vi "Main1.vi"() -> ()   [LabVIEW 2020]
uses:
  System.Windows.Forms
  Global_Variable/Global.vi
  Database/Global1.vi
  <userlib>/_MGI/Menu Building/MenuTypes/MenuStrip/MGI_MenuStrip.lvclass
  <userlib>/_MGI/Menu Building/MenuItemStatusChange/MGI_MenuItemStatusChange.lvclass
  Libraries/S7/S7.lvlib
panel:
  in  "Andon":enum32{"未选择", "缺料报警", "质量报警", "故障报警"}(radio)
  out "自动":bool
  out "结果显示":string
  in  "打印条码":bool caption="布尔"
  out "传感器值":dbl format="%#_4gN"
  out "上学状态":string="123"
  out "PLC":bool
  in  "菜单":refnum<k24>(container)
  out "试验计时":u16
  out "产品编号":string
  out "生产数量":i32
  out "合格数量":i32
  out "userStatus":string caption="用户状态"
  out "userName":string caption="用户名"
  out "connectionMode":string caption="联机类型"
  out "产品型号":string
  out "锁紧/开启":bool
  in  "更换产品":refnum<vi>
  out "提示信息":string
  out "错误":bool
  out "时间字符串":string
  out "日期字符串":string
  # "中间轴装配"
  # "装配工艺"
  # "上序状态"
  # "检测结果："
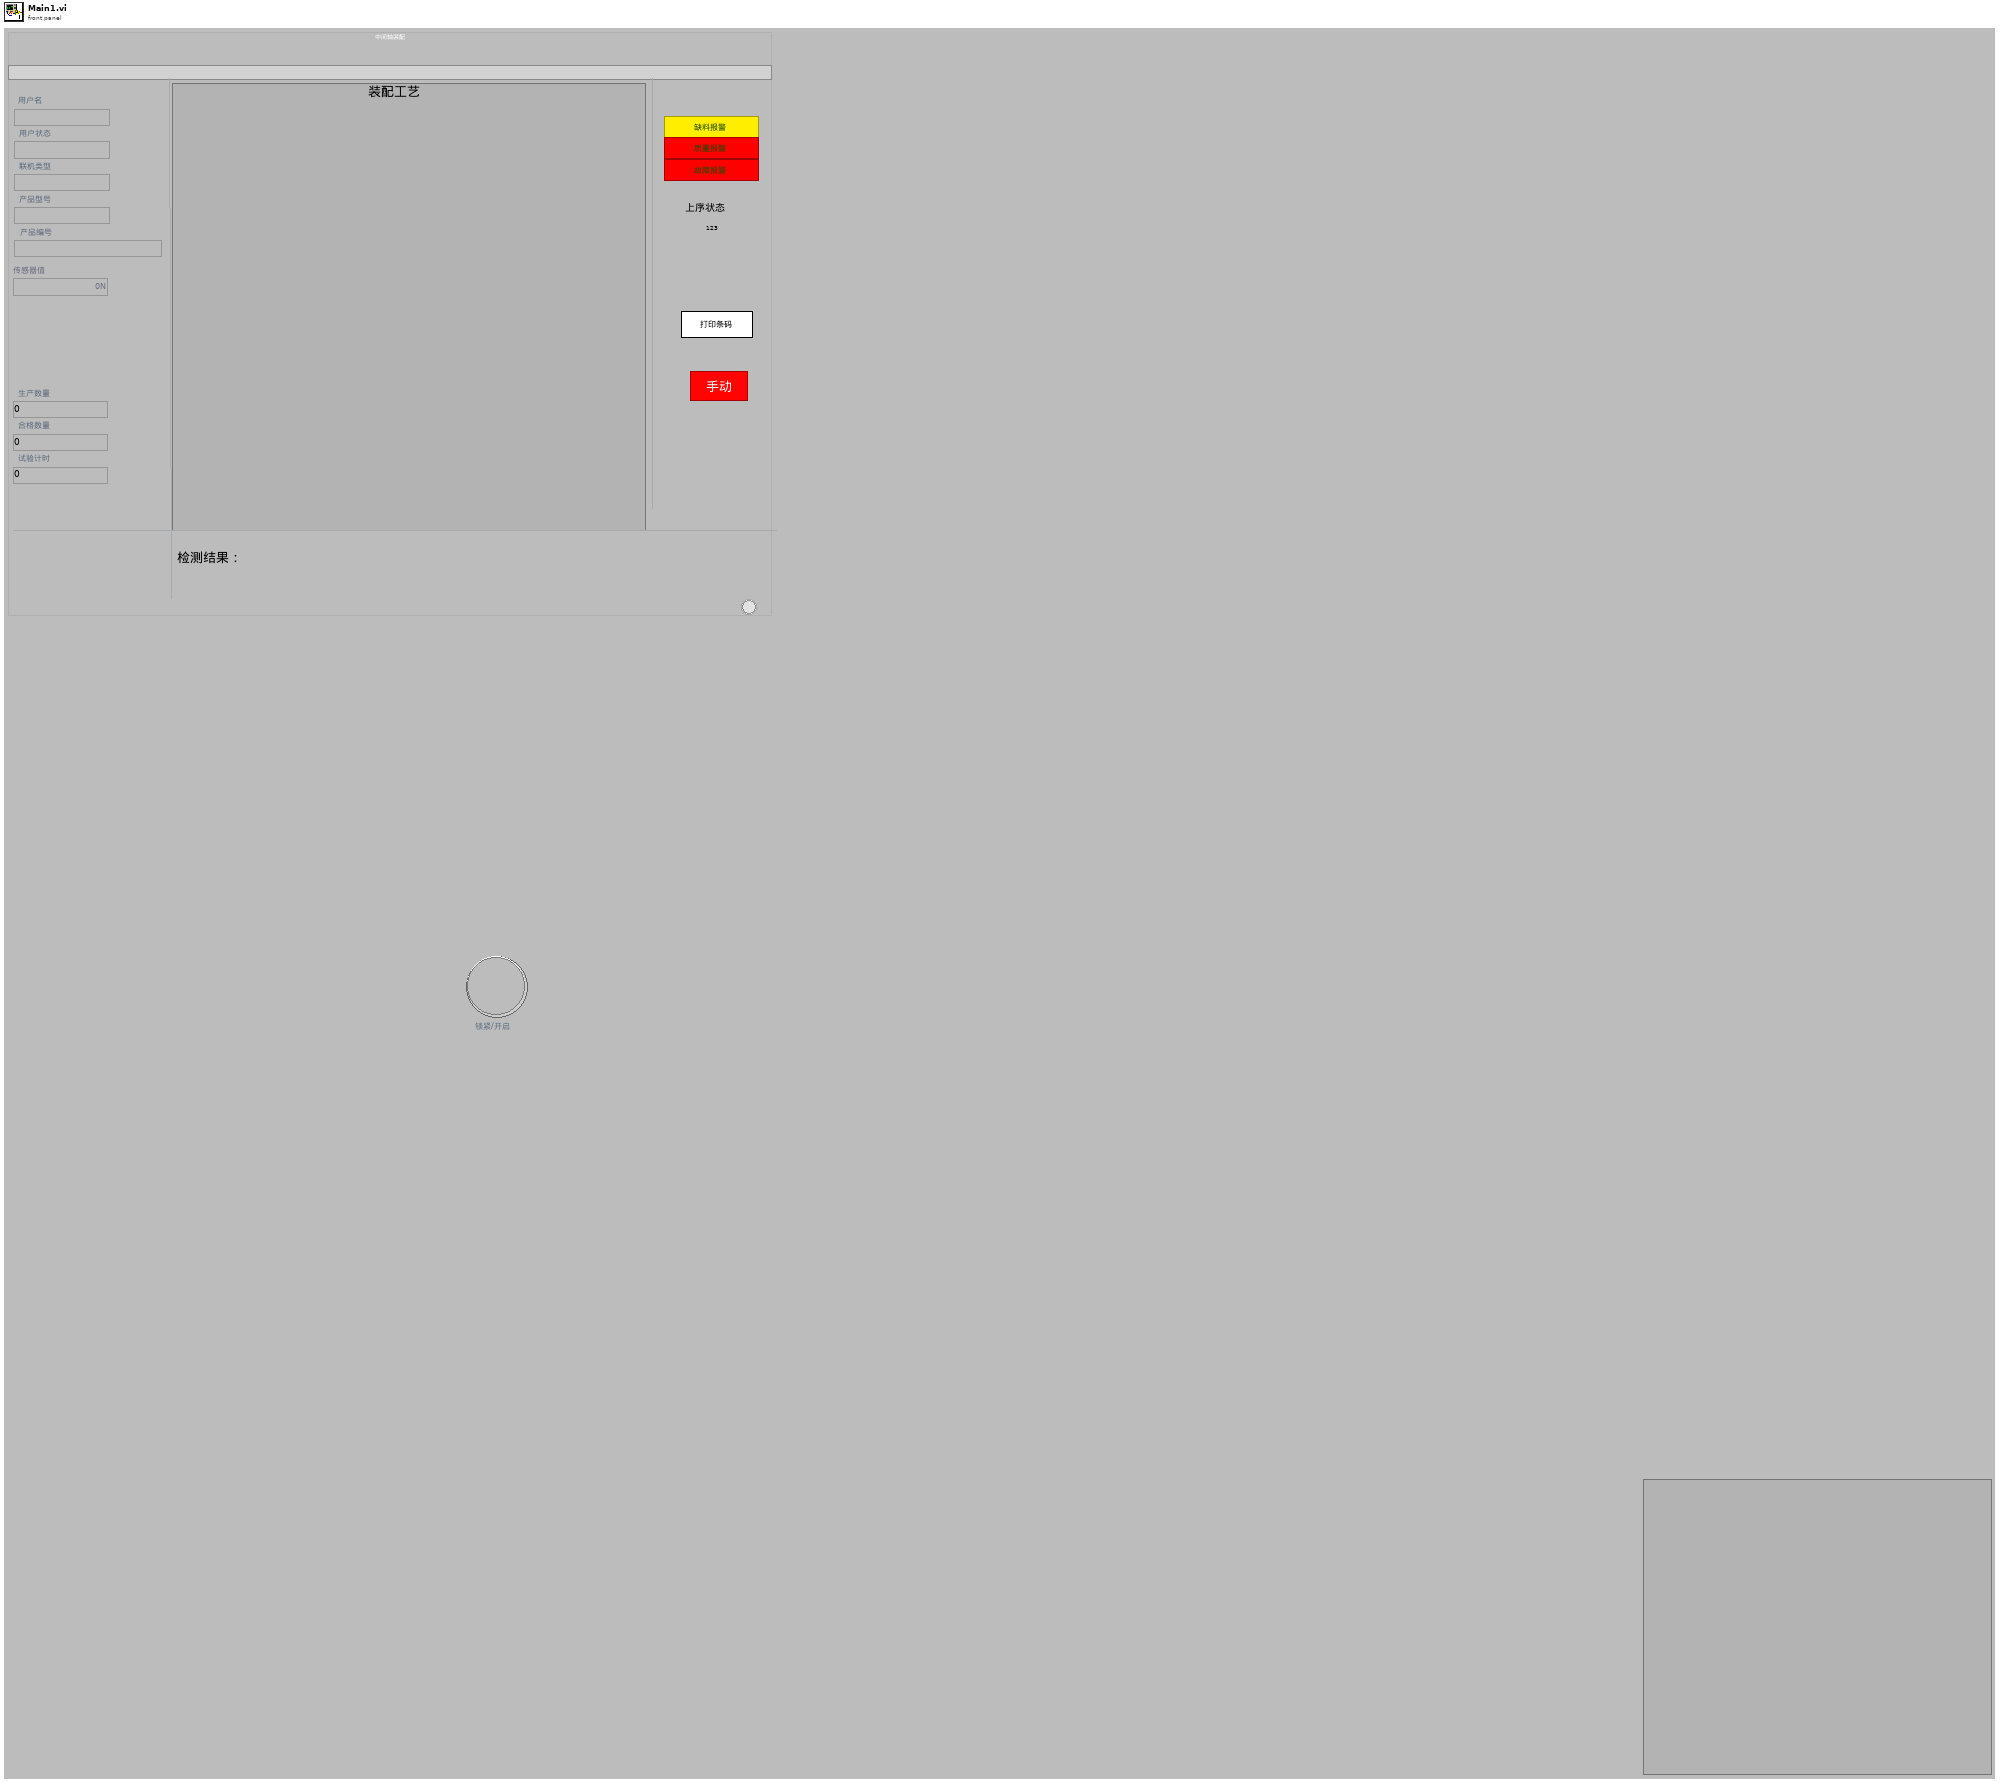
[diagram p1: front panel]
types:
  T1 = typedef "S7.lvlib/Broadcast Events--cluster.ctl" = cluster{"Module Did Init":refnum<user-event>, "Status Updated":refnum<user-event>, "Error Reported":refnum<user-event>, "Module Did Stop":refnum<user-event>, "Update Module Execution Status":refnum<user-event>}
  T2 = enum32{"Invalid", "Standard", "Closed", "Hidden", "Minimized", "Maximized"}
  T3 = cluster{"设备名称":string, "操作人员":string, "设备状态":enum16{"设备离线", "设备正常", "设备缺料", "设备故障", "质量报警"}, "附加信息":string}
  T4 = enum32{"invalid app kind", "Development System", "Run Time System", "Student Edition", "Embedded LabVIEW", "Evaluation", "Custom"}
  T5 = cluster{"扭矩":sgl, "输入移载位移":sgl, "工装移载位移":sgl, "输入编码位移":sgl, "输入扭矩":sgl, "输出扭矩(小)":sgl, "输出扭矩(大)":sgl, "吸收电流":sgl}
  T6 = cluster{"用户编号":string, "用户名":string, "用户密码(密文)":string, "用户权限":string}
  T7 = cluster{"Core":cluster{"Current VI Reference":refnum<vi>, "Close Panel on Exit?":bool}, "Your Boolean data":bool, "Your string data":string}
  T8 = enum32{"Bad", "Idle", "Run top level", "Running"}
  T9 = cluster{"Current VI Reference":refnum<vi>, "Close Panel on Exit?":bool}
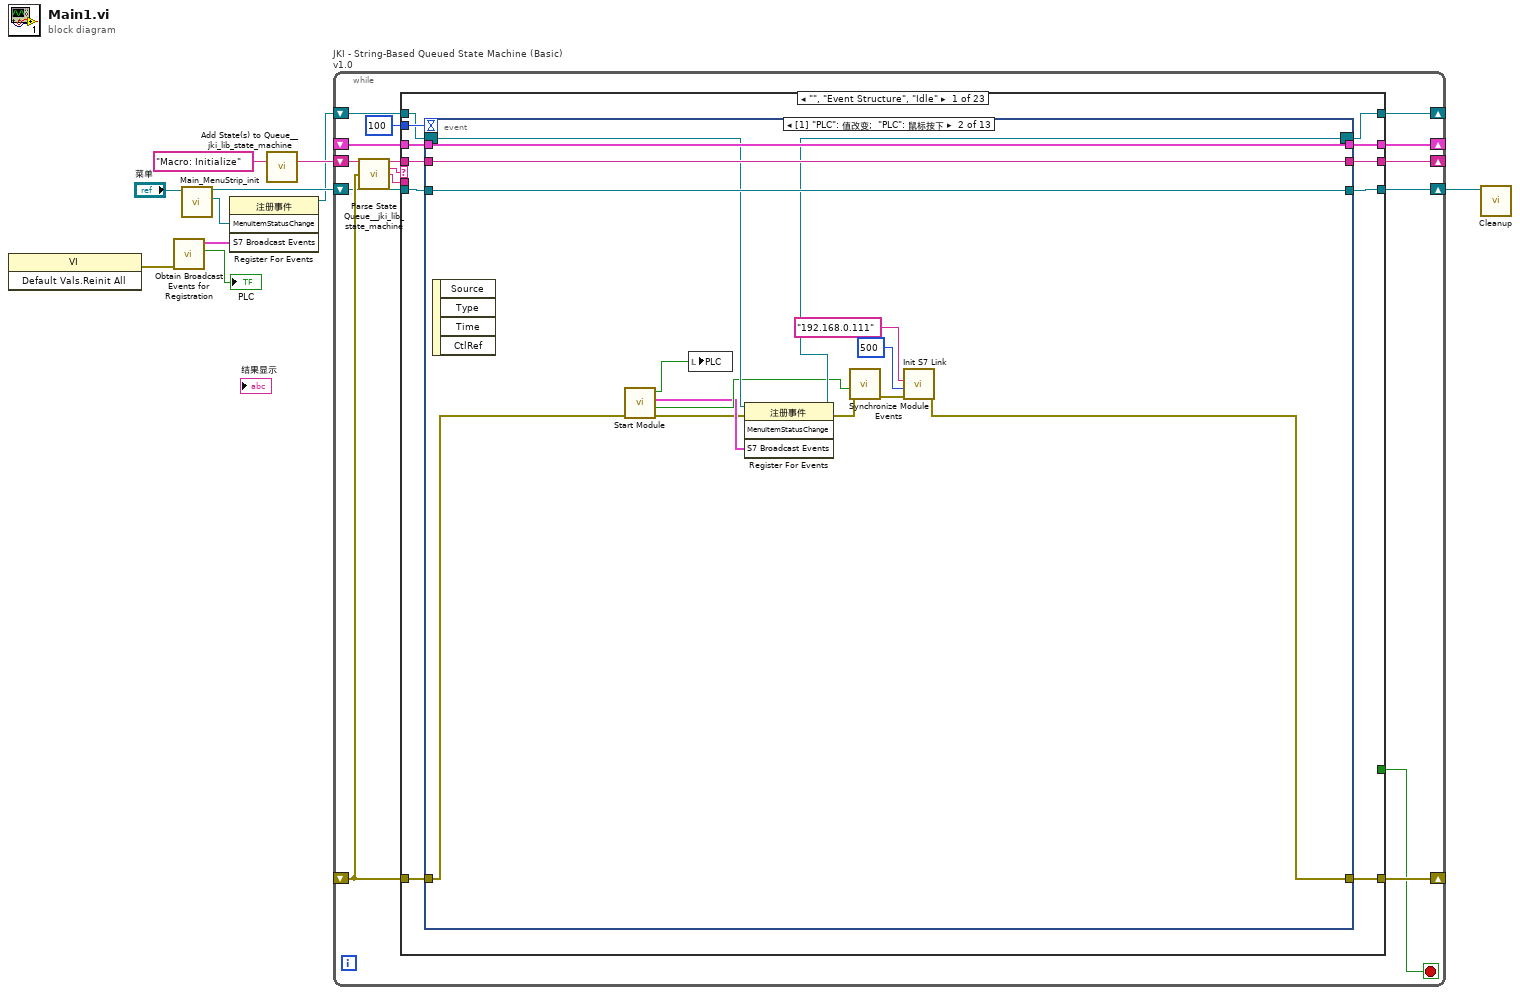
[diagram p0: block diagram]
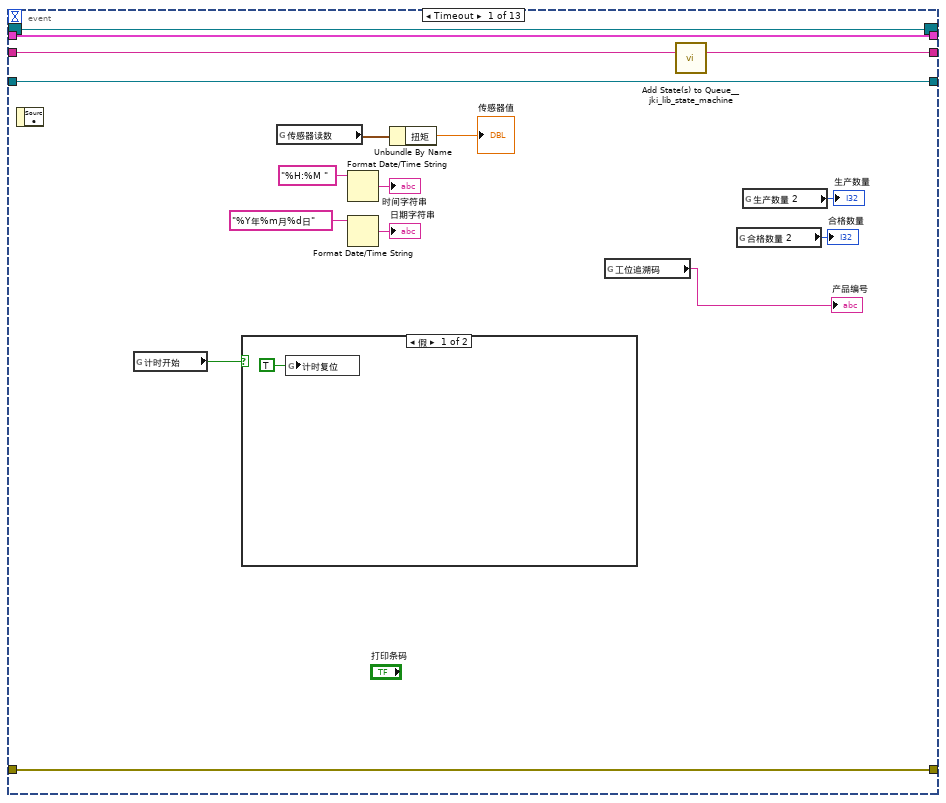
[diagram p2: hidden frame]
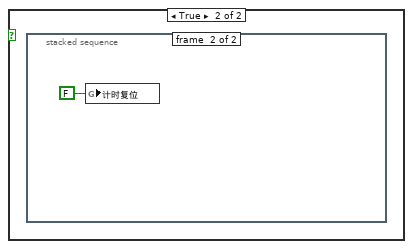
[diagram p3: hidden frame]
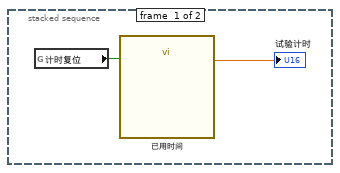
[diagram p4: hidden frame]
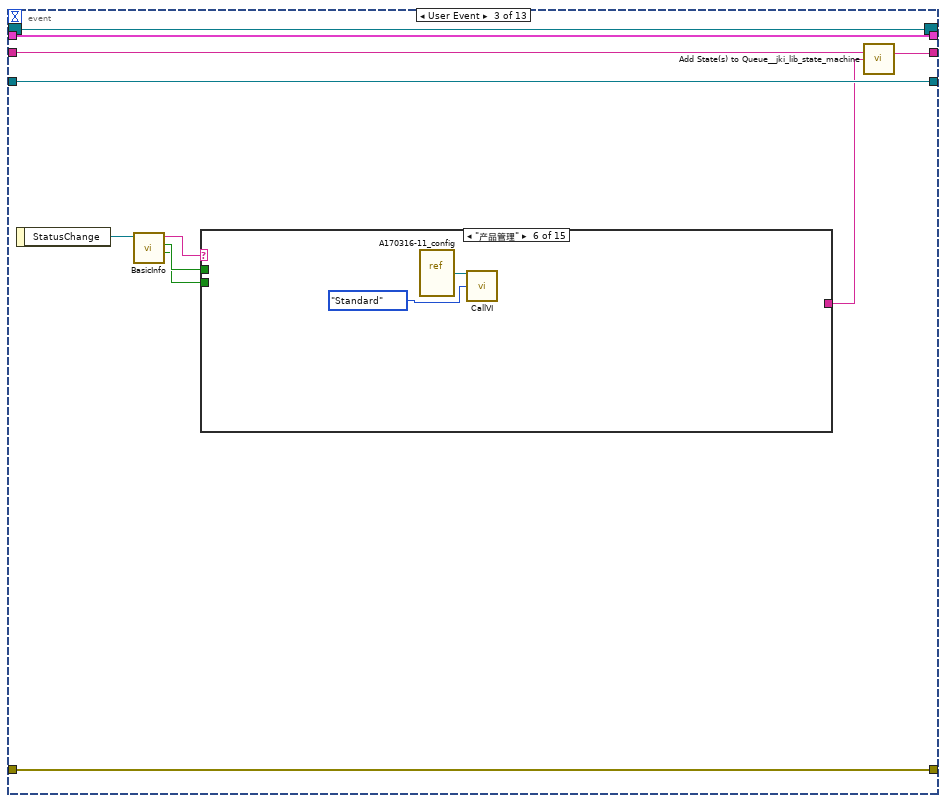
[diagram p5: hidden frame]
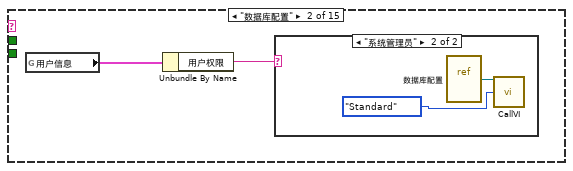
[diagram p7: hidden frame]
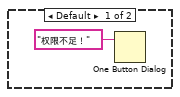
[diagram p8: hidden frame]
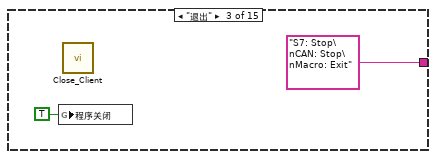
[diagram p9: hidden frame]
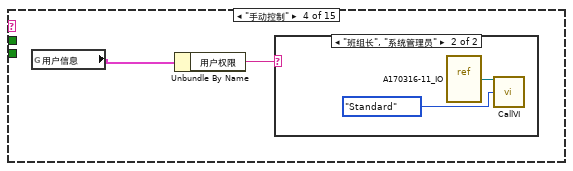
[diagram p10: hidden frame]
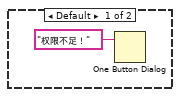
[diagram p11: hidden frame]
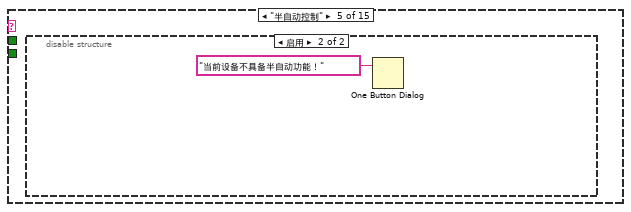
[diagram p12: hidden frame]
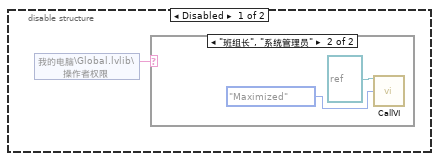
[diagram p13: hidden frame]
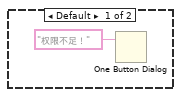
[diagram p14: hidden frame]
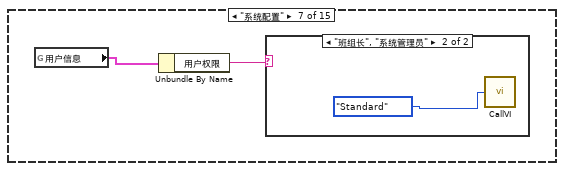
[diagram p15: hidden frame]
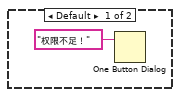
[diagram p16: hidden frame]
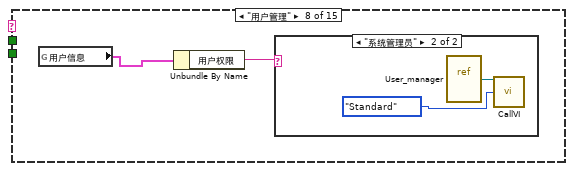
[diagram p17: hidden frame]
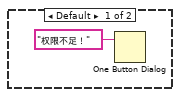
[diagram p18: hidden frame]
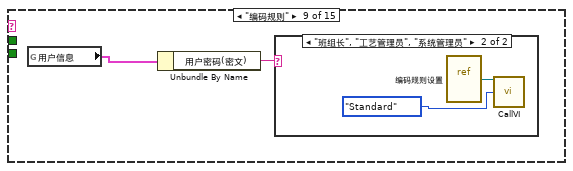
[diagram p19: hidden frame]
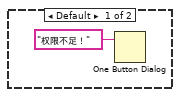
[diagram p20: hidden frame]
diagram:
  n1 = invoke class="VI" method="Default Vals.Reinit All"() -> (error out=w3:errorcluster)  [unwired: 3 in, 2 out]
  n2 = call "Obtain Broadcast Events for Registration.vi"("error in (no error)"=w3) -> ("Already running?"=→"PLC":bool, "S7 Broadcast Events"=w5:T1)  [unwired: 8 in, 1 out]
  n3 = call "Main_MenuStrip_init.vi"("MenuStrip"="菜单") -> ("MenuItemStatusChange"=w2:refnum<user-event>, "Menu out"=w7:refnum<class "MGI_MenuStrip.lvclass">)  [unwired: 9 in]
  n4 = register-events(w2, w5) -> (reference out=w1:refnum<event-registration>)  [unwired: 2 in, 1 out]
  n5 = call <vilib>:"Add State(s) to Queue__jki_lib_state_machine.vi"("State(s) in (\"\")"="Macro: Initialize") -> ("States Out"=w10:string)  [unwired: 14 in]
  n6 = while "JKI - String-Based Queued State Machine (Basic) v1.0" {
    shift-right: [w19] -> _
    shift-left: _ -> [w18]
    shift-right: [w21] -> _
    shift-left: _ -> [w16]
    shift-right: [w20] -> _
    shift-left: w10 -> [w22]
    shift-right: [w14] -> w6
    shift-left: w7 -> [w15]
    shift-right: [w12] -> _
    shift-left: w1 -> [w11]
    stop <- w13 stop-if-true
    n7 = call <vilib>:"Parse State Queue__jki_lib_state_machine.vi"("State Queue"=w22, "Error In (no error)"=w16) -> ("Remaining States"=w24:string, "Current State"=w25:string, "Arguments"=w23:string)  [unwired: 11 in]
    n8 = case shown="\"\", \"Event Structure\", \"Idle\"" w25 {
      selector: w25 -> [_ _ w242 _ _ _ _ _ _ _ _ _ _ _ _ _ _ _ _ _ _ _ _]
      tunnel: w24 -> [w36 w239 w246 w266 w274 w281 w287 w291 w297 w303 w324 w333 w344 w352 w358 w365 w392 w422 w430 w443 w471 w478 w490]
      tunnel: w23 -> [_ _ _ _ _ _ _ _ _ _ _ _ _ _ _ _ _ _ w425 w437 _ _ _]
      tunnel: w18 -> [w34 w236 w244 w257 w271 w279 w284 w292 w300 w306 w327 w330 _ w347 w355 w363 w390 w419 w428 w439 w468 w475 w487]
      tunnel: [w33 w237 w248 w263 errorcluster {"status"=FALSE, "code"=0, "source"=""} ("error out") w278 w285 w289 w295 w302 w323 w331 w341 w348 w356 w362 w388 w420 w426 w440 w469 w476 w488] -> w21
      tunnel: w16 -> [w32 w237 w247 w263 w270 w278 w285 w289 w296 w302 w323 w331 w341 w349 w356 w359 w388 w420 w427 w441 w469 w476 w488]
      tunnel: [w35 w238 w245 w265 w273 w280 w286 w291 w298 w304 w325 w332 w343 w351 w357 w364 w391 w421 w429 w442 w470 w477 w489] -> w20
      tunnel: [w31 w236 w244 w264 w271 w279 w284 w292 w300 w306 w327 w330 w342 w347 w355 w363 w390 w419 w428 w439 w468 w475 w487] -> w19
      tunnel: 100 ("Timeout") -> [w30 _ _ _ _ _ _ _ _ _ _ _ _ _ _ _ _ _ _ _ _ _ _]
      tunnel: w15 -> [w29 w235 w241 w254 w268 w277 w283 w290 w299 w305 w326 w329 w335 w346 w354 w361 w389 w418 w424 w436 w467 w473 w480]
      tunnel: [w28 w235 w241 w254 w268 w277 w283 w290 w299 w305 w326 w329 w335 w346 w354 w361 w389 w418 w424 w436 w467 w473 w480] -> w14
      tunnel: [_ _ _ _ _ TRUE _ _ _ _ _ _ _ _ _ _ _ _ _ _ _ _ _] -> w13
      tunnel: [w26 w234 w240 w253 w267 w275 w282 w293 w294 w301 w322 w328 w336 w345 w353 w360 w387 w415 w423 w435 w466 w472 w479] -> w12
      tunnel: w11 -> [w27 w234 w240 w253 w267 w275 w282 w293 w294 w301 w322 w328 w336 w345 w353 w360 w387 w415 w423 w435 w466 w472 w479]
      frame "", "Event Structure", "Idle" {
        n9 = event shown="[1] \"PLC\": 值改变;  \"PLC\": 鼠标按下" {
          selector: w27 -> [w41 w66 w72 w137 w144 w151 w158 w173 w188 w190 w197 w206 _]
          dyn-events: [w41 w65 w72 w137 w144 w151 w158 w173 w188 w190 w197 w206 _] -> w26
          timeout: w30 -> [_ _ _ _ _ _ _ _ _ _ _ _ _]
          tunnel: w36 -> [w52 w70 w81 w138 w145 w154 w161 w170 w186 w194 w204 w208 w228]
          tunnel: [w51 w70 w79 w139 w146 w155 w162 w171 w186 w195 w203 w209 w228] -> w35
          tunnel: w34 -> [w50 w71 w80 w141 w149 w156 w163 w172 w187 w196 w201 w211 w229]
          tunnel: [w42 w67 w82 w142 w147 w152 w164 w168 w184 w193 w202 w210 w226] -> w33
          tunnel: w32 -> [w42 w68 w82 w142 w147 w152 w165 w168 w184 w193 w202 w210 w226]
          tunnel: [w50 w71 w80 w141 w149 w156 w163 w172 w187 w196 w201 w211 w229] -> w31
          tunnel: w29 -> [w40 w69 w75 w140 w148 w153 w160 w169 w185 _ _ _ w227]
          tunnel: [w40 w69 w75 w140 w148 w153 w160 w169 w185 _ _ _ w227] -> w28
          event Timeout {
            n10 = event-data() -> ()  [unwired: 1 in, 1 out]
            n11 = global read "Global.vi" "计时开始"() -> (w43:bool)
            n12 = case shown="假" w43 {
              frame False {
                n13 = global write "Global.vi" "计时复位"(TRUE ("计时复位")) -> ()
              }
              frame True {
                n14 = stacked-sequence {
                  frame #0 {
                    n15 = global read "Global.vi" "计时复位"() -> (w54:bool)
                    n16 = call "已用时间"("Reset"=w54) -> ("Elapsed Time (s)"=→"试验计时":dbl)  [unwired: 11 in, 7 out]
                  }
                  frame #1 {
                    n17 = global write "Global.vi" "计时复位"(FALSE ("计时复位")) -> ()
                  }
                }
              }
            }
            n18 = global read "Global.vi" "传感器读数"() -> (w38:T5)
            n19 = Format Date/Time String(time format string (%c)="%H:%M ") -> (date/time string=→"时间字符串":string)  [unwired: 2 in]
            n20 = Format Date/Time String(time format string (%c)="%Y年%m月%d日") -> (date/time string=→"日期字符串":string)  [unwired: 2 in]
            n21 = Unbundle By Name(w38) -> ("扭矩"=→"传感器值":sgl)
            n22 = global read "Global1.vi" "工位追溯码"() -> (→"产品编号":string)
            n23 = call <vilib>:"Add State(s) to Queue__jki_lib_state_machine.vi"("State(s) in (\"\")"=w52) -> ("States Out"=w51:string)  [unwired: 14 in]
            n24 = global read "Global.vi" "合格数量 2"() -> (→"合格数量":i32)
            n25 = global read "Global.vi" "生产数量 2"() -> (→"生产数量":i32)
          }
          event "PLC": Value Change; "PLC": Mouse Down {
            n26 = event-data() -> ()  [unwired: 1 in, 4 out]
            n27 = call "Start Module.vi"("error in (no error)"=w68) -> ("error out"=w61:errorcluster, "Wait for Event Sync?"=w64:bool, "S7 Broadcast Events"=w63:T1, "Module Was Already Running?"=w62:bool)  [unwired: 7 in]
            n28 = local write "PLC"(w62) -> ()
            n29 = register-events(reference=w66, error in=w61, w63) -> (reference out=w65:refnum<event-registration>, error out=w60:errorcluster)  [unwired: 1 in]
            n30 = call "Synchronize Module Events.vi"("error in (no error)"=w60, "Wait for Event Sync?"=w64) -> ("error out"=w57:errorcluster)  [unwired: 9 in]
            n31 = call "Init S7 Link.vi"("error in (no error)"=w57, "超时"=500, "IP"="192.168.0.111") -> ("error out"=w67:errorcluster)  [unwired: 8 in]
          }
          event User Event {
            n32 = event-data() -> ("StatusChange"=w73:refnum<class "MGI_MenuItemStatusChange.lvclass">)  [unwired: 1 in]
            n33 = call <userlib>:"BasicInfo.vi"("MGI_MenuItemStatusChange in"=w73) -> ("Enabled?"=w76:bool, "Checked?"=w77:bool, "Tag"=w78:string)  [unwired: 7 in, 1 out]
            n34 = case shown="\"产品管理\"" w78 {
              tunnel: w77 -> [_ _ _ _ _ _ _ _ _ _ _ _ _ _ _]
              tunnel: w76 -> [_ _ _ _ _ _ _ _ _ _ _ _ _ _ _]
              tunnel: [_ _ "S7: Stop\nCAN: Stop\nMacro: Exit" _ _ _ _ _ _ _ _ _ _ _ _] -> w74
              frame "假", Default {
              }
              frame "数据库配置" {
                n35 = global read "Global1.vi" "用户信息"() -> (w83:T6)
                n36 = Unbundle By Name(w83) -> ("用户权限"=w84:string)
                n37 = case shown="\"系统管理员\"" w84 {
                  frame Default {
                    n38 = One Button Dialog(message="权限不足！" ("消息")) -> ()  [unwired: 1 in, 1 out]
                  }
                  frame "系统管理员" {
                    n39 = vi-ref "数据库配置.vi"() -> (w87:refnum<vi>)
                    n40 = call "CallVI.vi"("VI引用"=w87, "状态"=T2."Standard") -> ()  [unwired: 11 in, 3 out]
                  }
                }
              }
              frame "退出" {
                n41 = global write "Global.vi" "程序关闭"(TRUE ("程序关闭")) -> ()
                n42 = call "Close_Client.vi"() -> ()  [unwired: 12 in]
              }
              frame "手动控制" {
                n43 = global read "Global1.vi" "用户信息"() -> (w90:T6)
                n44 = Unbundle By Name(w90) -> ("用户权限"=w91:string)
                n45 = case shown="\"班组长\", \"系统管理员\"" w91 {
                  frame Default {
                    n46 = One Button Dialog(message="权限不足！" ("消息")) -> ()  [unwired: 1 in, 1 out]
                  }
                  frame "班组长", "系统管理员" {
                    n47 = vi-ref "A170316-11_IO.vi"() -> (w94:refnum<vi>)
                    n48 = call "CallVI.vi"("VI引用"=w94, "状态"=T2."Standard") -> ()  [unwired: 11 in, 3 out]
                  }
                }
              }
              frame "半自动控制" {
                n49 = disable-structure shown="启用" {
                  frame Disabled {
                    n50 = shared-variable "我的电脑\\Global.lvlib\\操作者权限"() -> (w95:string)  [unwired: 1 in, 1 out]
                    n51 = case shown="\"班组长\", \"系统管理员\"" w95 {
                      frame Default {
                        n52 = One Button Dialog(message="权限不足！" ("消息")) -> ()  [unwired: 1 in, 1 out]
                      }
                      frame "班组长", "系统管理员" {
                        n53 = call "CallVI.vi"("VI引用"=refnum<vi> refnum, "状态"=T2."Maximized") -> ()  [unwired: 11 in, 3 out]
                      }
                    }
                  }
                  frame Enabled {
                    n54 = One Button Dialog(message="当前设备不具备半自动功能！" ("消息")) -> ()  [unwired: 1 in, 1 out]
                  }
                }
              }
              frame "产品管理" {
                n55 = vi-ref "A170316-11_config.vi"() -> (w101:refnum<vi>)
                n56 = call "CallVI.vi"("VI引用"=w101, "状态"=T2."Standard") -> ()  [unwired: 11 in, 3 out]
              }
              frame "系统配置" {
                n57 = global read "Global1.vi" "用户信息"() -> (w102:T6)
                n58 = Unbundle By Name(w102) -> ("用户权限"=w103:string)
                n59 = case shown="\"班组长\", \"系统管理员\"" w103 {
                  frame Default {
                    n60 = One Button Dialog(message="权限不足！" ("消息")) -> ()  [unwired: 1 in, 1 out]
                  }
                  frame "班组长", "系统管理员" {
                    n61 = call "CallVI.vi"("状态"=T2."Standard") -> ()  [unwired: 12 in, 3 out]
                  }
                }
              }
              frame "用户管理" {
                n62 = global read "Global1.vi" "用户信息"() -> (w106:T6)
                n63 = Unbundle By Name(w106) -> ("用户权限"=w107:string)
                n64 = case shown="\"系统管理员\"" w107 {
                  frame Default {
                    n65 = One Button Dialog(message="权限不足！" ("消息")) -> ()  [unwired: 1 in, 1 out]
                  }
                  frame "系统管理员" {
                    n66 = vi-ref "User_manager.vi"() -> (w110:refnum<vi>)
                    n67 = call "CallVI.vi"("VI引用"=w110, "状态"=T2."Standard") -> ()  [unwired: 11 in, 3 out]
                  }
                }
              }
              frame "编码规则" {
                n68 = global read "Global1.vi" "用户信息"() -> (w111:T6)
                n69 = Unbundle By Name(w111) -> ("用户密码(密文)"=w112:string)
                n70 = case shown="\"班组长\", \"工艺管理员\", \"系统管理员\"" w112 {
                  frame Default {
                    n71 = One Button Dialog(message="权限不足！" ("消息")) -> ()  [unwired: 1 in, 1 out]
                  }
                  frame "班组长", "工艺管理员", "系统管理员" {
                    n72 = vi-ref "编码规则设置.vi"() -> (w115:refnum<vi>)
                    n73 = call "CallVI.vi"("VI引用"=w115, "状态"=T2."Standard") -> ()  [unwired: 11 in, 3 out]
                  }
                }
              }
              frame "易损件管理" {
                n74 = vi-ref "易损件管理.vi"() -> (w117:refnum<vi>)
                n75 = call "CallVI.vi"("VI引用"=w117, "状态"=T2."Standard") -> ()  [unwired: 11 in, 3 out]
              }
              frame "物料批次管理" {
                n76 = vi-ref "批次管理.vi"() -> (w119:refnum<vi>)
                n77 = call "CallVI.vi"("VI引用"=w119, "状态"=T2."Standard") -> ()  [unwired: 11 in, 3 out]
              }
              frame "报表" {
                n78 = call "文件对话框"("start path"=path "D:/report", "prompt"="打开报表", "pattern (all files)"="*.doc;*.docx", "pattern label"="Word 文档") -> ("selected path"=w120:path, "error out"=w121:errorcluster)  [unwired: 8 in, 2 out]
                n79 = case shown="无错误" w121 {
                  selector: w121 -> [w127 w129]
                  tunnel: w120 -> [w128 _]
                  frame No Error {
                    w126 = 1 items=["Normal", "Maximize", "Minimize"] ("cpubbs_WindowState")
                    n80 = call "Open_Word.vi"("File Path"=w128, "cpubbs_WindowState"=w126, "错误输入（无错误）"=w127) -> ()  [unwired: 12 in, 1 out]
                  }
                  frame Error {
                    n81 = call <vilib>:"Clear Errors.vi"("error in (no error)"=w129) -> ()  [unwired: 5 in, 2 out]
                  }
                }
              }
              frame "报警信息" {
                n82 = vi-ref "报警信息.vi"() -> (w131:refnum<vi>)
                n83 = call "CallVI.vi"("VI引用"=w131, "状态"=T2."Standard") -> ()  [unwired: 11 in, 3 out]
              }
              frame "关于" {
                n84 = vi-ref "About.vi"() -> (w133:refnum<vi>)
                n85 = call "CallVI.vi"("VI引用"=w133, "状态"=T2."Standard") -> ()  [unwired: 11 in, 3 out]
              }
              frame "操作演示" {
                n86 = call <vilib>:"Application Directory.vi"() -> ("Application Directory"=w136:path)
                n87 = Build Path(base path=w136, name or relative path="操作演示" ("名称或相对路径")) -> (appended path=w135:path)
                n88 = call "自动播放ppt.vi"("路径"=w135) -> ()  [unwired: 10 in, 1 out]
              }
            }
            n89 = call <vilib>:"Add State(s) to Queue__jki_lib_state_machine.vi"("State(s) in (\"\")"=w81, "State(s) at Back (\"\")"=w74) -> ("States Out"=w79:string)  [unwired: 13 in]
          }
          event User Event {
            n90 = event-data() -> ("Init?"=w143:bool)  [unwired: 1 in, 1 out]
            n91 = local write "PLC"(w143) -> ()
            n92 = call <vilib>:"Add State(s) to Queue__jki_lib_state_machine.vi"("State(s) in (\"\")"=w138) -> ("States Out"=w139:string)  [unwired: 14 in]
          }
          event User Event {
            n93 = event-data() -> ("Running?"=w150:bool)  [unwired: 1 in]
            n94 = local write "PLC"(w150) -> ()
            n95 = call <vilib>:"Add State(s) to Queue__jki_lib_state_machine.vi"("State(s) in (\"\")"=w145) -> ("States Out"=w146:string)  [unwired: 14 in]
          }
          event User Event {
            n96 = event-data() -> ()  [unwired: 1 in, 7 out]
            n97 = local write "PLC"(FALSE ("PLC")) -> ()
            n98 = call <vilib>:"Add State(s) to Queue__jki_lib_state_machine.vi"("State(s) in (\"\")"=w154) -> ("States Out"=w155:string)  [unwired: 14 in]
          }
          event User Event {
            n99 = event-data() -> ("Error"=w166:errorcluster)  [unwired: 1 in]
            n100 = Merge Errors(w166, w165) -> (w164:errorcluster)
            n101 = call <vilib>:"Add State(s) to Queue__jki_lib_state_machine.vi"("State(s) in Front (\"\")"="S7: Initialize\nIdle", "State(s) in (\"\")"=w161) -> ("States Out"=w162:string)  [unwired: 13 in]
          }
          event "自动": Mouse Down {
            n102 = event-data() -> ()  [unwired: 1 in, 8 out]
            n103 = local read "自动"() -> (w167:bool)
            n104 = case shown="假" w167 {
              frame False {
                n105 = shared-variable "我的电脑\\A17031611.lvlib\\设备状态"() -> (w174:i16)  [unwired: 1 in, 1 out]
                n106 = case shown="5" w174 {
                  frame 0, Default {
                    n107 = One Button Dialog(message="请复位！" ("消息")) -> ()  [unwired: 1 in, 1 out]
                  }
                  frame 5 {
                    n108 = vi-ref "A170316-11_Auto.vi"() -> (w176:refnum<vi>)
                    n109 = invoke class="VI" method="Ctrl Val.Set"(reference=w176, "Control Name"="STEP" ("控件名"), "Value"="初始化" ("控件名")) -> ()  [unwired: 2 in, 5 out]
                  }
                }
              }
              frame True {
                n110 = Two Button Dialog(message="确定要退出自动？" ("消息")) -> (T button?=w179:bool)  [unwired: 2 in]
                n111 = case shown="真" w179 {
                  frame False {
                  }
                  frame True {
                    n112 = vi-ref "A170316-11_Auto.vi"() -> (w183:refnum<vi>)
                    n113 = invoke class="VI" method="Ctrl Val.Set"(reference=w183, "Control Name"="STEP" ("控件名"), "Value"="手动" ("控件名")) -> ()  [unwired: 2 in, 5 out]
                  }
                }
              }
            }
            n114 = call <vilib>:"Add State(s) to Queue__jki_lib_state_machine.vi"("State(s) in (\"\")"=w170) -> ("States Out"=w171:string)  [unwired: 14 in]
          }
          event "打印条码": Value Change {
            n115 = event-data() -> ()  [unwired: 1 in, 6 out]
            n116 = global read "Global.vi" "产品型号"() -> (w189:string)
            n117 = case shown="\"R92A\"" w189 {
              frame Default {
                n118 = call "Barcodeprint.vi"() -> ()  [unwired: 12 in]
              }
              frame "R92A" {
                n119 = call "BarcodeprintR92A.vi"() -> ()  [unwired: 12 in]
              }
              frame "R092B" {
                n120 = call "BarcodeprintR92A.vi"() -> ()  [unwired: 12 in]
              }
            }
          }
          event "错误": Mouse Down {
            n121 = event-data() -> ()  [unwired: 1 in, 8 out]
            n122 = vi-ref "报警信息.vi"() -> (w192:refnum<vi>)
            n123 = call "CallVI.vi"("VI引用"=w192, "状态"=T2."Standard") -> ()  [unwired: 11 in, 3 out]
            n124 = call <vilib>:"Add State(s) to Queue__jki_lib_state_machine.vi"("State(s) in (\"\")"=w194) -> ("States Out"=w195:string)  [unwired: 14 in]
          }
          event Panel Close? {
            n125 = event-data() -> ()  [unwired: 1 in, 1 out]
            n126 = global write "Global.vi" "程序关闭"(TRUE ("程序关闭")) -> ()
            n127 = call <vilib>:"Add State(s) to Queue__jki_lib_state_machine.vi"("State(s) in Front (\"\")"="S7: Stop\nMacro: Exit", "State(s) in (\"\")"=w204) -> ("States Out"=w203:string)  [unwired: 13 in]
            n128 = event-data("Discard?"=TRUE) -> ()  [unwired: 1 in, 1 out]
          }
          event "更换产品": Value Change {
            n129 = event-data() -> ("NewVal"=w207:refnum<vi>)  [unwired: 1 in, 5 out]
            n130 = stacked-sequence {
              tunnel: w207 -> [w213]
              tunnel: [w212] -> w205
              frame #0 {
                n131 = stacked-sequence {
                  tunnel: w213 -> [w216 _]
                  tunnel: [_ w217] -> w212
                  frame #0 {
                    n132 = control-ref of="子面板"() -> (w214:refnum<vi>)
                    n133 = global read "Global.vi" "产品型号"() -> (w215:string)
                    n134 = call "Call_SubPanal.vi"("VI引用句柄"=w216, "SubPnl引用句柄"=w214) -> ()  [unwired: 9 in, 1 out]
                    n135 = local write "产品型号"(w215) -> ()
                  }
                  frame #1 {
                    n136 = global read "Global.vi" "启用CAN"() -> (w218:bool)
                    n137 = case shown="真" w218 {
                      tunnel: ["CAN: Stop" "CAN: Stop\nIdle\nCAN: Start"] -> w217
                      frame False {
                      }
                      frame True {
                      }
                    }
                  }
                }
              }
            }
            n138 = call <vilib>:"Add State(s) to Queue__jki_lib_state_machine.vi"("State(s) in Front (\"\")"=w205, "State(s) in (\"\")"=w208) -> ("States Out"=w209:string)  [unwired: 13 in]
          }
          event "Andon": Value Change {
            n139 = event-data() -> ("NewVal"=w225:enum32{"未选择", "缺料报警", "质量报警", "故障报警"})  [unwired: 1 in]
            n140 = case shown="\"缺料报警\"" w225 {
              tunnel: [enum16{"设备离线", "设备正常", "设备缺料", "设备故障", "质量报警"}."设备正常" ("设备状态") enum16{"设备离线", "设备正常", "设备缺料", "设备故障", "质量报警"}."设备缺料" ("设备状态") enum16{"设备离线", "设备正常", "设备缺料", "设备故障", "质量报警"}."质量报警" ("设备状态") enum16{"设备离线", "设备正常", "设备缺料", "设备故障", "质量报警"}."设备故障" ("设备状态")] -> w223
              frame "未选择", Default {
              }
              frame "缺料报警" {
              }
              frame "质量报警" {
              }
              frame "故障报警" {
              }
            }
            n141 = local read "userName"() -> (w222:string)
            n142 = Bundle By Name(cluster=T3 {"设备名称"="中间轴装配", "操作人员"="", "设备状态"=enum."设备离线", "附加信息"=""} ("设备信息"), "操作人员"=w222, "设备状态"=w223) -> (w221:T3)
            n143 = call "Change_Client.vi"("设备信息"=w221) -> ()  [unwired: 10 in, 1 out]
          }
        }
      }
      frame "---------- Core ----------" {
        n144 = call <vilib>:"Add State(s) to Queue__jki_lib_state_machine.vi"("State(s) in (\"\")"=w239) -> ("States Out"=w238:string)  [unwired: 14 in]
      }
      frame Default {
        w251 = 42 items=["No error", "Argument error", "Memory is full", "Out of zone", "End of file", "File already open", "Generic file I/O error", "File not found", "File permission error", "Disk is full", "Duplicate path", "Too many files open", "System feature not enabled", "Resource file not found", "Cannot add resource", "Resource not found", "Image not found", "Image memory error", "Pen does not exist", "Config type invalid", "Config token not found", "Config parse error", "Config memory error", "Bad external code format", "Bad external code offset", "External code not present", "Null window", "Destroy window error", "Null menu", "Print aborted", "Bad print record", "Print driver error", "Windows error during printing", "Memory error during printing", "Print dialog error", "Generic print error", "Invalid device refnum", "Device not found", "Device parameter error", "Device unit error", "Cannot open device", "Device call aborted", "Generic error", "Cancelled by user", "Object ID too low", "Object ID too high", "Object not in heap", "Unknown heap", "Unknown object (invalid DefProc)", "Unknown object (DefProc not in table)", "Message out of range", "Invalid (null) method", "Unknown message", "Manager call not supported", "Bad address", "Network operation in progress", "Network operation timed out", "Connection is busy", "Network attribute not supported", "Network error", "Address in use", "System out of memory", "Connection aborted", "Connection refused", "Not connected", "Already connected", "Connection closed", "Initialization error (interapplication manager)", "Bad occurrence", "Wait on unbound occurrence handler", "Occurrence queue overflow", "Datalog type conflict", "Unused", "Unrecognized type (interapplication manager)", "Memory corrupt", "Failed to make temporary DLL", "Old CIN version", "Drag socket not found", "Failed to load drop-object", "Failed to register OLE object", "Failed to release OLE object", "Format specifier type mismatch", "Unknown format specifier", "Too few format specifiers", "Too many format specifiers", "Scan failed", "Newer CIN version", "Error converting to variant", "Runtime menu error", "Password tampered", "Variant attribute not found", "Incompatible variant data type", "Event data is not available", "Event Store is not present", "Occurrence is not found", "Event Queue is not created", "Event info is not available", "Refnum passed is NULL", "Error retrieving Class GUID", "Error retrieving CoClass GUID", "Error retrieving TypeLib GUID.", "Bad built application magic bytes.", "Specific driver is different from the specific driver associated with the Logical Name.", "There is no session opened to the class driver.", "Max Error", "MAX - Error with config objects", "MAX - Error loading configuration", "MAX - Group not supported"]
        # "Current State"
        n145 = Format Into String(format string="Software Exception: Unhandled State \"%s\"." ("message"), error in=w247, w242) -> (resulting string=w250:string, error out=w249:errorcluster)  [unwired: 1 in]
        n146 = call <vilib>:"Error Cluster From Error Code.vi"("show call chain? (False)"=TRUE, "error in (no error)"=w249, "error message (\"\")"=w250, "error code (0)"=w251) -> ("error out"=w248:errorcluster)  [unwired: 5 in]
        n147 = call <vilib>:"Add State(s) to Queue__jki_lib_state_machine.vi"("State(s) in (\"\")"=w246) -> ("States Out"=w245:string)  [unwired: 14 in]
      }
      frame "Initialize Core Data" {
        # "originally closed?"
        # "exe?"
        n148 = property class="VI"() -> ("Front Panel.Open"=w262:bool)  [unwired: 2 in, 2 out]
        n149 = property class="App"() -> ("App.Kind"=w261:T4)  [unwired: 2 in, 2 out]
        n150 = control-ref of="Current VI Reference"() -> (w255:refnum<vi>)
        n151 = Not(x=w262) -> (.not. x?=w259:bool)
        n152 = Equal?(x=w261, y=T4."Run Time System" ("Application:Kind")) -> (x = y?=w258:bool)
        n153 = Or(x=w259, y=w258) -> (x .or. y?=w256:bool)
        n154 = Bundle By Name(cluster=w257, "Core.Current VI Reference"=w255, "Core.Close Panel on Exit?"=w256) -> (w264:T7)
        n155 = call <vilib>:"Add State(s) to Queue__jki_lib_state_machine.vi"("State(s) in (\"\")"=w266) -> ("States Out"=w265:string)  [unwired: 14 in]
      }
      frame "Error Handler" {
        n156 = call <vilib>:"General Error Handler.vi"("error in (no error)"=w270) -> ()  [unwired: 10 in, 5 out]
        n157 = call <vilib>:"Add State(s) to Queue__jki_lib_state_machine.vi"("State(s) in Front (\"\")"="/* Post Error States", "State(s) in (\"\")"=w274) -> ("States Out"=w273:string)  [unwired: 13 in]
      }
      frame "Exit" {
        n158 = call <vilib>:"Add State(s) to Queue__jki_lib_state_machine.vi"("State(s) in (\"\")"=w281) -> ("States Out"=w280:string)  [unwired: 14 in]
        n159 = Quit LabVIEW() -> ()  [unwired: 1 in]
      }
      frame "--------- Library --------" {
        n160 = call <vilib>:"Add State(s) to Queue__jki_lib_state_machine.vi"("State(s) in (\"\")"=w287) -> ("States Out"=w286:string)  [unwired: 14 in]
      }
      frame "S7: Initialize" {
        n161 = property on="PLC" class="Bool (严格)"("Val(Sgnl)"=FALSE ("值(信号)")) -> ()  [unwired: 2 in, 2 out]
      }
      frame "S7: Stop" {
        n162 = call "Stop Module.vi"("error in (no error)"=w296) -> ("error out"=w295:errorcluster)  [unwired: 10 in]
        n163 = call <vilib>:"Add State(s) to Queue__jki_lib_state_machine.vi"("State(s) in (\"\")"=w297) -> ("States Out"=w298:string)  [unwired: 14 in]
      }
      frame "CAN: Start" {
        n164 = while {
          stop <- w308 stop-if-true
          n165 = vi-ref "CAN.vi"() -> (w312:refnum<vi>)
          n166 = call "CallVI.vi"("VI引用"=w312, "状态"=T2."Hidden") -> ("VI引用输出"=w307:refnum<vi>, "错误输出"=w309:errorcluster)  [unwired: 11 in, 1 out]
          n167 = property class="VI"(reference=w307, error in=w309) -> ("Exec.State"=w310:T8)  [unwired: 2 out]
          n168 = case shown="\"Run top level\"" w310 {
            tunnel: [w313 TRUE TRUE] -> w308
            frame "Bad", Default {
              n169 = Two Button Dialog(message="CAN卡打开失败！" ("消息"), 1:"重试" ("F按钮名称（“取消”）"), 2:"忽略" ("T按钮名称（“确定”）")) -> (T button?=w313:bool)
            }
            frame "Run top level" {
            }
            frame "Running" {
            }
          }
        }
        n170 = call <vilib>:"Add State(s) to Queue__jki_lib_state_machine.vi"("State(s) in (\"\")"=w303) -> ("States Out"=w304:string)  [unwired: 14 in]
      }
      frame "CAN: Stop" {
        n171 = vi-ref "CAN.vi"() -> (w321:refnum<vi>)
        n172 = invoke class="VI" method="Ctrl Val.Set"(reference=w321, "Control Name"="Stop" ("控件名"), "Value"=TRUE) -> ()  [unwired: 2 in, 5 out]
        n173 = call <vilib>:"Add State(s) to Queue__jki_lib_state_machine.vi"("State(s) in (\"\")"=w324) -> ("States Out"=w325:string)  [unwired: 14 in]
      }
      frame "---------- Data ----------" {
        n174 = call <vilib>:"Add State(s) to Queue__jki_lib_state_machine.vi"("State(s) in (\"\")"=w333) -> ("States Out"=w332:string)  [unwired: 14 in]
      }
      frame "Data: Initialize" {
        w338 = T9 {"Current VI Reference"=refnum, "Close Panel on Exit?"=FALSE}  # Core
        w340 = TRUE  # Your Boolean data
        w339 = ""  # Your string data
        n175 = global write "Global.vi" "程序关闭"(FALSE ("程序关闭")) -> ()
        n176 = global write "Global.vi" "计时开始"(FALSE ("计时结束")) -> ()
        n177 = Bundle("Core"=w338, "Your Boolean data"=w340, "Your string data"=w339) -> (w342:T7)  [unwired: 1 in]
        n178 = call <vilib>:"Add State(s) to Queue__jki_lib_state_machine.vi"("State(s) in (\"\")"=w344) -> ("States Out"=w343:string)  [unwired: 14 in]
      }
      frame "Data: Cleanup" {
        n179 = Unbundle By Name(w347) -> ("Core.Current VI Reference"=w350:refnum<vi>)
        n180 = Close Reference(reference=w350, error in (no error)=w349) -> (error out=w348:errorcluster)
        n181 = call <vilib>:"Add State(s) to Queue__jki_lib_state_machine.vi"("State(s) in (\"\")"=w352) -> ("States Out"=w351:string)  [unwired: 14 in]
      }
      frame "---------- UI ----------" {
        # "Do not put any code in this frame.\n(It is a separator no-op. You can make a copy of this frame to create a new UI frame)"
        n182 = call <vilib>:"Add State(s) to Queue__jki_lib_state_machine.vi"("State(s) in (\"\")"=w358) -> ("States Out"=w357:string)  [unwired: 14 in]
      }
      frame "UI: Initialize" {
        n183 = disable-structure shown="禁用" {
          frame Disabled {
            n184 = vi-ref "A170316-11_Auto.vi"() -> (w368:refnum<vi>)
            n185 = invoke class="VI" method="Ctrl Val.Set"(reference=w368, "Control Name"="STEP" ("控件名"), "Value"="自动" ("控件名")) -> ()  [unwired: 2 in, 5 out]
          }
          frame Enabled {
          }
        }
        n186 = disable-structure shown="启用" {
          disable-tunnel: [w375 _] -> w362
          disable-tunnel: w359 -> [w373 _]
          frame Enabled {
            n187 = vi-ref "A170316-11_Auto.vi"() -> (w374:refnum<vi>)
            n188 = property class="VI"(reference=w374) -> (reference out=w372:refnum<vi>, "FP.State"=w371:T2)  [unwired: 1 in, 1 out]
            n189 = case shown="\"Standard\", 默认" w371 {
              tunnel: w373 -> [w381 w383]
              tunnel: w372 -> [w382 w384]
              tunnel: [w380 w384] -> w369
              tunnel: [w379 w383] -> w370
              frame "Standard", Default {
                n190 = invoke class="VI" method="FP.Close"(reference=w382, error in=w381) -> (reference out=w380:refnum<vi>, error out=w379:errorcluster)  [unwired: 1 in, 1 out]
              }
              frame "Invalid", "Closed" {
              }
            }
            n191 = invoke on="子面板" class="SubPnl" method="Insert VI"(error in=w370, "VI Ref"=w369) -> (error out=w378:errorcluster)  [unwired: 2 in, 3 out]
            n192 = invoke class="VI" method="Run VI"(reference=w369, error in=w378, "Wait until done"=FALSE ("结束前等待"), "Auto Dispose Ref"=TRUE ("自动销毁引用")) -> (error out=w375:errorcluster)  [unwired: 1 in, 4 out]
          }
          frame Disabled {
            n193 = vi-ref "Auto.vi"() -> (w386:refnum<vi>)
            n194 = call "CallVI.vi"("VI引用"=w386, "状态"=T2."Maximized") -> ()  [unwired: 11 in, 3 out]
          }
        }
        n195 = call <vilib>:"Add State(s) to Queue__jki_lib_state_machine.vi"("State(s) in (\"\")"=w365) -> ("States Out"=w364:string)  [unwired: 14 in]
      }
      frame "UI: Init" {
        n196 = stacked-sequence {
          tunnel: w388 -> [_ _ _ _ _]
          frame #0 {
            n197 = vi-ref "状态读取.vi"() -> (w394:refnum<vi>)
            n198 = call "CallVI.vi"("VI引用"=w394, "状态"=T2."Hidden") -> ()  [unwired: 11 in, 3 out]
            n199 = property on="上学状态" class="Str"("Text.BGColor"=u32 16777216 ("文本.文本颜色:背景色")) -> ()  [unwired: 2 in, 2 out]
          }
          frame #1 {
            n200 = global write "Global.vi" "程序关闭"(FALSE ("程序关闭")) -> ()
            n201 = control-ref of="结果显示"() -> (w396:refnum<vi>)
            n202 = control-ref of="上学状态"() -> (w397:refnum<vi>)
            n203 = global write "Global.vi" "结果显示"(w396) -> ()
            n204 = global write "Global.vi" "前序显示字"(w397) -> ()
          }
          frame #2 {
            w407 = 0
            n205 = shared-variable "我的电脑\\Global.lvlib\\总成追溯码"("   " ("工位追溯码")) -> ()  [unwired: 1 in, 1 out]
            n206 = global read "Global.vi" "前序显示字"() -> (w402:refnum<vi>)
            n207 = global write "Global.vi" "生产数量 2"(w407) -> ()
            n208 = global write "Global.vi" "合格数量 2"(w407) -> ()
            n209 = global read "Global1.vi" "用户信息"() -> (w400:T6)
            n210 = global read "Global1.vi" "联机模式"() -> (w399:enum16{"单机", "联网"})
            n211 = property class="Str"(reference=w402, "Value"="" ("值")) -> ()  [unwired: 1 in, 2 out]
            n212 = Unbundle By Name(w400) -> ("用户名"=→"userName":string, "用户权限"=→"userStatus":string)
            n213 = case shown="\"联网\"" w399 {
              tunnel: ["联网" ("connectionMode") "单机" ("connectionMode")] -> w408
              frame "联网" {
              }
              frame "单机", Default {
              }
            }
            "connectionMode" <- w408
            "产品型号" <- "" ("产品型号")
          }
          frame #3 {
            n214 = control-ref of="自动"() -> (w411:refnum<vi>)
            n215 = control-ref of="提示信息"() -> (w413:refnum<vi>)
            n216 = control-ref of="错误"() -> (w414:refnum<vi>)
            n217 = control-ref of="更换产品"() -> (w412:refnum<vi>)
            n218 = global write "Global.vi" "提示信息"(w413) -> ()
            n219 = global write "Global.vi" "程序自动"(w411) -> ()
            n220 = global write "Global.vi" "报警图标"(w414) -> ()
            n221 = global write "Global.vi" "更换产品"(w412) -> ()
          }
          frame #4 {
            n222 = call "Start_Client.vi"() -> ()  [unwired: 12 in]
          }
        }
        n223 = call <vilib>:"Add State(s) to Queue__jki_lib_state_machine.vi"("State(s) in (\"\")"=w392) -> ("States Out"=w391:string)  [unwired: 14 in]
      }
      frame "UI: Config" {
        n224 = vi-ref "A170316-11_config.vi"() -> (w417:refnum<vi>)
        n225 = call "CallVI.vi"("VI引用"=w417, "状态"=T2."Standard") -> ()  [unwired: 11 in, 3 out]
        n226 = call <vilib>:"Add State(s) to Queue__jki_lib_state_machine.vi"("State(s) in (\"\")"=w422) -> ("States Out"=w421:string)  [unwired: 14 in]
      }
      frame "UI: Cursor Set" {
        # "Argument"
        n227 = case shown="\"Idle\", 默认" w425 {
          tunnel: w427 -> [w432 w434]
          tunnel: [w431 w433] -> w426
          frame "Idle", Default {
            n228 = call <vilib>:"Unset Busy.vi"("error in (no error)"=w432) -> ("error out"=w431:errorcluster)  [unwired: 10 in]
          }
          frame "Busy" {
            n229 = call <vilib>:"Set Busy.vi"("error in (no error)"=w434) -> ("error out"=w433:errorcluster)  [unwired: 9 in, 1 out]
          }
        }
        n230 = call <vilib>:"Add State(s) to Queue__jki_lib_state_machine.vi"("State(s) in (\"\")"=w430) -> ("States Out"=w429:string)  [unwired: 14 in]
      }
      frame "UI: Front Panel State" {
        # "Argument"
        n231 = Unbundle By Name(w439) -> ("Core.Current VI Reference"=w438:refnum<vi>)
        n232 = case shown="\"Close\"" w437 {
          tunnel: w441 -> [w447 w460]
          tunnel: [w449 w461] -> w440
          tunnel: w438 -> [w448 w458]
          frame "Open", Default {
            n233 = property class="VI"(reference=w448, error in=w447) -> (reference out=w445:refnum<vi>, error out=w446:errorcluster, "Front Panel.Open"=w444:bool)
            n234 = case shown="假" w444 {
              tunnel: [w452 w455] -> w449
              tunnel: w446 -> [w451 w455]
              tunnel: w445 -> [w450 _]
              frame False {
                n235 = invoke class="VI" method="FP.Open"(reference=w450, error in=w451, "Activate"=TRUE, "State"=T2."Standard") -> (error out=w452:errorcluster)  [unwired: 1 in, 4 out]
              }
              frame True {
              }
            }
          }
          frame "Close" {
            n236 = property class="VI"(reference=w458, error in=w460) -> (reference out=w457:refnum<vi>, error out=w459:errorcluster, "Front Panel.Open"=w456:bool)
            n237 = case shown="真" w456 {
              tunnel: [w462 w465] -> w461
              tunnel: w459 -> [w462 w464]
              tunnel: w457 -> [_ w463]
              frame False {
              }
              frame True {
                n238 = invoke class="VI" method="FP.Close"(reference=w463, error in=w464) -> (error out=w465:errorcluster)  [unwired: 1 in, 2 out]
              }
            }
          }
        }
        n239 = call <vilib>:"Add State(s) to Queue__jki_lib_state_machine.vi"("State(s) in (\"\")"=w443) -> ("States Out"=w442:string)  [unwired: 14 in]
      }
      frame "---------- Macro ----------" {
        n240 = call <vilib>:"Add State(s) to Queue__jki_lib_state_machine.vi"("State(s) in (\"\")"=w471) -> ("States Out"=w470:string)  [unwired: 14 in]
      }
      frame "Macro: Initialize" {
        n241 = call <vilib>:"Add State(s) to Queue__jki_lib_state_machine.vi"("State(s) in Front (\"\")"="Data: Initialize\nInitialize Core Data\nS7: Initialize\nIdle\nUI: Init\nUI: Front Panel State >> Open\nUI: Initialize\nUI: Config", "State(s) in (\"\")"=w478) -> ("States Out"=w477:string)  [unwired: 13 in]
      }
      frame "Macro: Exit" {
        n242 = Unbundle By Name(w487) -> ("Core.Close Panel on Exit?"=w486:bool)
        n243 = Select(t="UI: Front Panel State >> Close", s=w486, f="") -> (s? t:f=w483:string)
        n244 = call <vilib>:"Add State(s) to Queue__jki_lib_state_machine.vi"("State(s) in (\"\")"=w483, "State(s) at Back (\"\")"="Data: Cleanup\nExit") -> ("States Out"=w481:string)  [unwired: 13 in]
        n245 = call <vilib>:"Add State(s) to Queue__jki_lib_state_machine.vi"("State(s) in Front (\"\")"=w481, "State(s) in (\"\")"=w490) -> ("States Out"=w489:string)  [unwired: 13 in]
      }
    }
  }
  n246 = call-dynamic "Cleanup.vi"("MenuStrip in"=w6) -> ()  [unwired: 10 in, 1 out]
